vi "画箭头.vi"(0 "Image 2":T1(plugin-control)=refnum, 5 "距离":dbl, 7 "Rectangle":T3={"Left"=1066, "Top"=296, "Right"=344, "Bottom"=354, "Rotation"=45.0} {"Rotation" format="%.2f"; "Left" scale=0.0..1024.0; "Right" scale=0.0..1024.0}, 9 "abgek":dbl, 11 "error in (no error)":errorcluster caption="错误输入（无错误）", 12 "long":sgl=15.0, 13 "Color 2":u32(colorbox)=16711680) -> (4 "Image":T1(plugin-control), 15 "error out":errorcluster)   [LabVIEW 2017]
uses:
  <vilib>/Analysis/coordinate.llb/2D Cartesian Coordinate Shift (Array).vi
  <vilib>/Analysis/coordinate.llb/2D Cartesian Coordinate Rotation (Array).vi
  <vilib>/Analysis/NI_AALPro.lvlib
panel:
  out "下":dbl
  out "上":dbl
  in  "Width":u32=23
  out "添加的数组":T2[](array[typedef]) {"Y" format="%.2f"; "X" format="%.2f"}
  in  "Color":u32(colorbox)=16711680
  out "MiddleEndPoint":T2={"X"=892.0, "Y"=1299.75} {"Y" format="%.2f"; "X" format="%.2f"}
  out "MiddleStartPoint":T2={"X"=892.0, "Y"=1159.25} {"Y" format="%.2f"; "X" format="%.2f"}
  out "EndPoint":T2={"X"=892.0, "Y"=1370.0} {"Y" format="%.2f"; "X" format="%.2f"}
  out "StartPoint":T2={"X"=892.0, "Y"=1089.0} {"Y" format="%.2f"; "X" format="%.2f"}
  in  "sss":i32=30
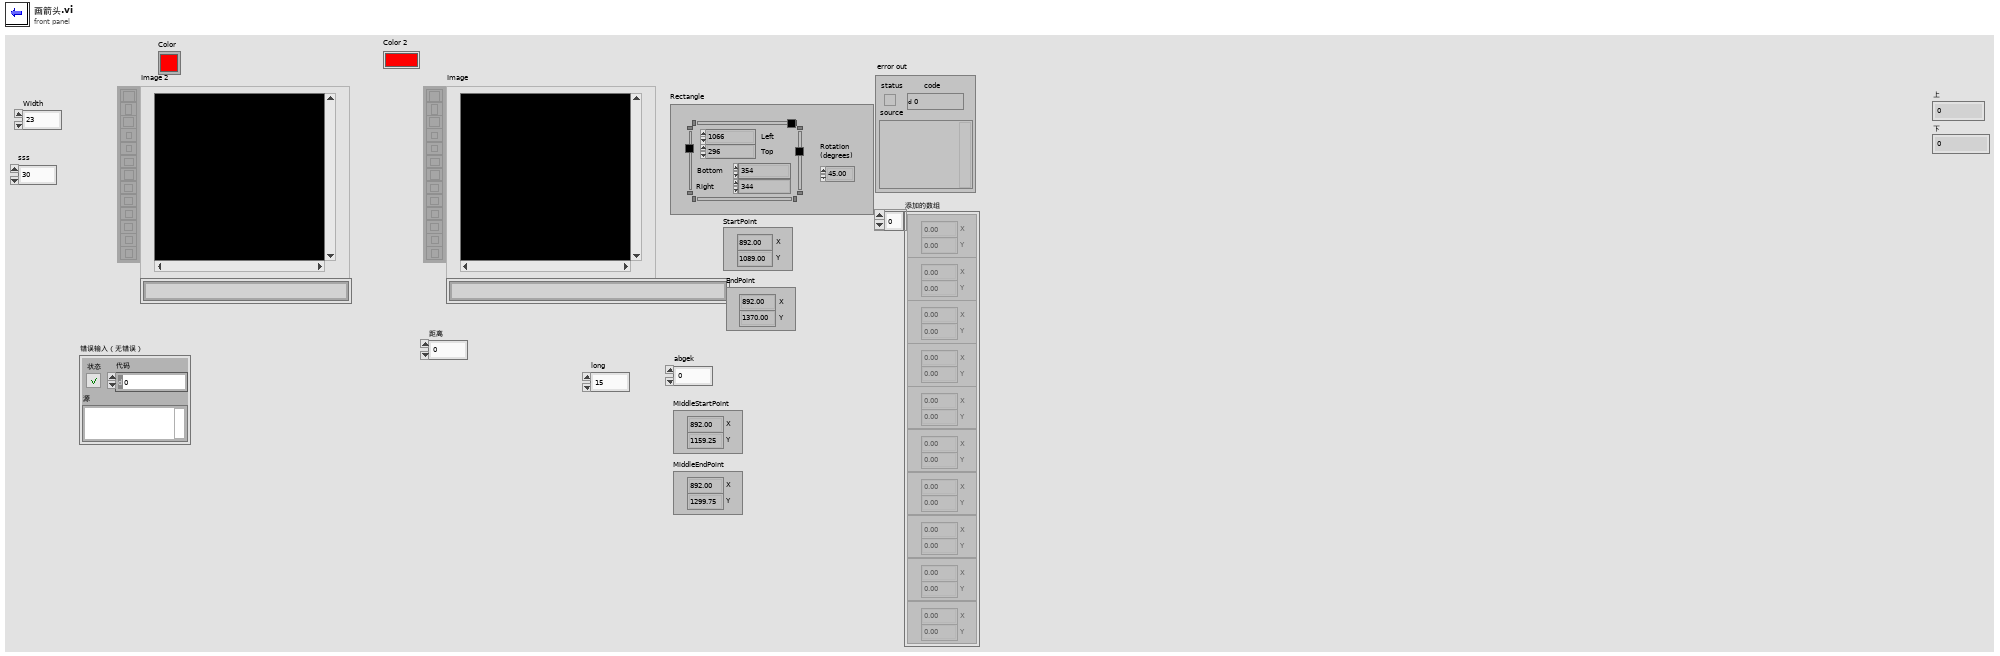
[diagram p1: front panel]
types:
  T1 = typedef "IMAQ Image.ctl" = refnum<image>
  T2 = typedef "IMAQ Point" = cluster{"X":sgl, "Y":sgl}
  T3 = typedef "IMAQ Rectangle" = cluster{"Left":i32, "Top":i32, "Right":i32, "Bottom":i32, "Rotation":dbl}
  T4 = cluster{"Desired Font (Application)":enum16{"User-specified Font", "Application Font", "System Font", "Dialog Font"}, "[User-specified Font]":cluster{"Font Name":string, "Size":i16, "Strikeout?":bool, "Italic?":bool, "Underline?":bool, "Outline?":bool, "Shadow?":bool, "Bold?":bool, "Rotation Angle":dbl}, "Horizontal Alignment":i16, "Vertical Alignment":i16}
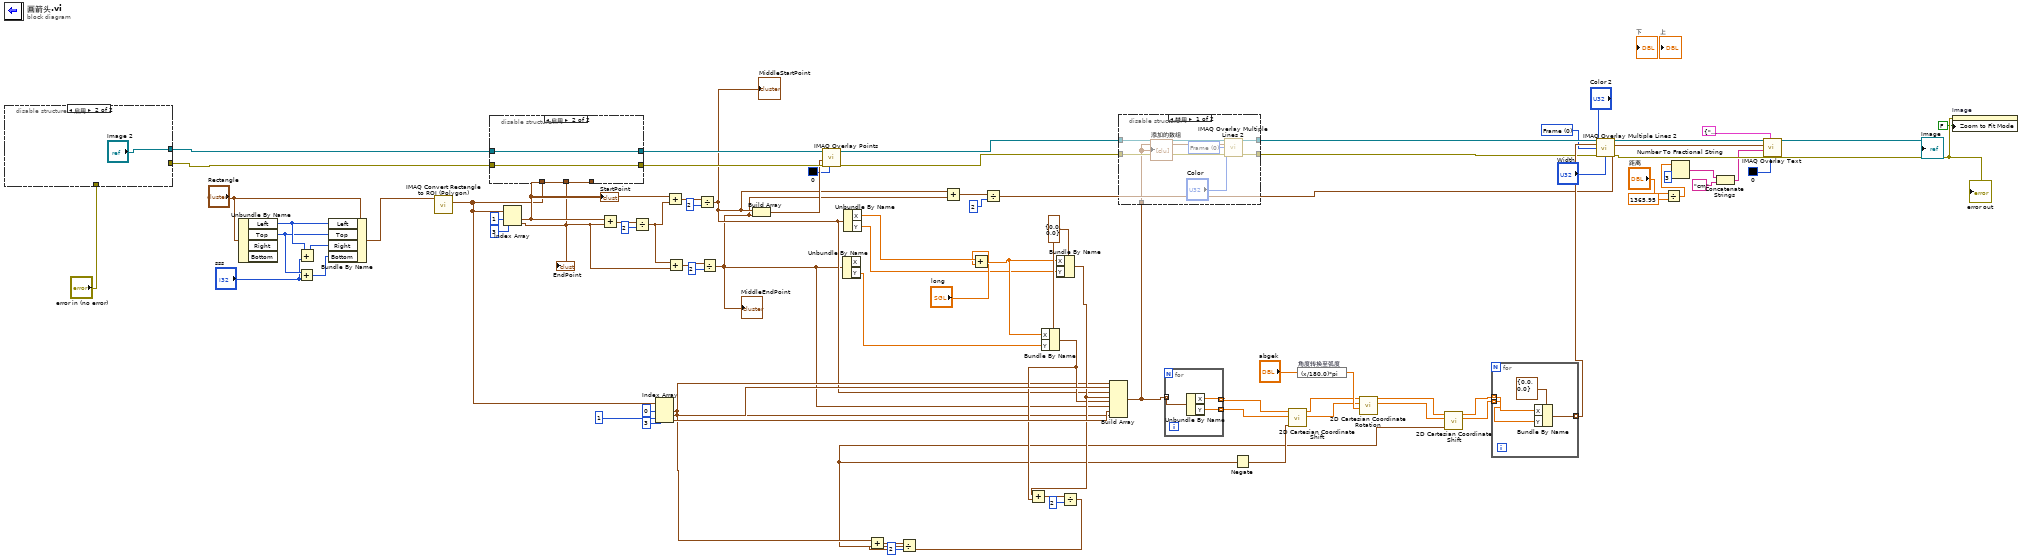
[diagram p0: block diagram]
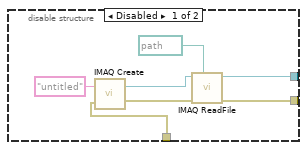
[diagram p2: hidden frame]
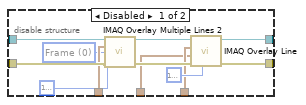
[diagram p4: hidden frame]
diagram:
  w32 = u32 0 items=["Frame", "Fill"] ("Drawing Mode (Frame)")
  w54 = T2 {"X"=0.0, "Y"=0.0} ("元素")
  n1 = disable-structure shown="启用" {
    disable-tunnel: [w87 "Image 2"] -> w17
    disable-tunnel: [w86 _] -> w16
    disable-tunnel: "error in (no error)" -> [w85 _]
    frame Disabled {
      n2 = call "IMAQ Create"("Image Name"="untitled", "error in (no error)"=w85) -> ("New Image"=w89:T1, "error out"=w90:errorcluster)  [unwired: 3 in]
      n3 = call "IMAQ ReadFile"("File Path"=path "C:/Users/Lenovo/Desktop/PowerLine Inspect System/微信图片_20181113103336.bmp", "error in (no error)"=w90, "Image"=w89) -> ("error out"=w86:errorcluster, "Image Out"=w87:T1)  [unwired: 4 in, 3 out]
    }
    frame Enabled {
    }
  }
  n4 = Unbundle By Name("Rectangle") -> ("Left"=w82:i32, "Top"=w80:i32)  [unwired: 2 out]
  n5 = Add(x=w80, y="sss") -> (x+y=w78:i32)
  n6 = Add(x=w82, y="sss") -> (x+y=w81:i32)
  n7 = Bundle By Name(cluster="Rectangle", "Left"=w82, "Top"=w80, "Right"=w81, "Bottom"=w78) -> (w83:T3)
  n8 = call "IMAQ Convert Rectangle to ROI (Polygon)"("Rectangle"=w83) -> ("Rectangle Points"=w57:T2[])  [unwired: 7 in, 2 out]
  n9 = Index Array(array=w57, index #1=1 ("索引"), index #2=3 ("索引")) -> (element #1=w70:T2, element #2=w66:T2)
  "StartPoint" <- w70
  "EndPoint" <- w66
  n10 = disable-structure shown="启用" {
    disable-tunnel: w17 -> [w103 w106]
    disable-tunnel: w16 -> [w102 w105]
    disable-tunnel: [w101 w106] -> w77
    disable-tunnel: w70 -> [w98 _]
    disable-tunnel: w66 -> [w97 _]
    disable-tunnel: [w96 w105] -> w64
    disable-tunnel: w57 -> [w95 _]
    frame Disabled {
      w94 = u32 0 items=["Frame", "Fill"] ("Drawing Mode (Frame)")
      n11 = call "IMAQ Overlay Multiple Lines 2"("Image"=w103, "Line End Points"=w95, "Drawing Mode (Frame)"=w94, "Color"=u32 16777238, "error in (no error)"=w102) -> ("Image Out"=w104:T1, "error out"=w100:errorcluster)  [unwired: 9 in]
      n12 = call "IMAQ Overlay Line"("Color"=u32 16777238, "error in (no error)"=w100, "End Point"=w97, "Start Point"=w98, "Image"=w104) -> ("error out"=w96:errorcluster, "Image Out"=w101:T1)  [unwired: 5 in]
    }
    frame Enabled {
    }
  }
  n13 = Add(x=w70, y=w66) -> (x+y=w74:T2)
  n14 = Divide(x=w74, y=2) -> (x/y=w67:T2)
  n15 = Index Array(array=w57, index #1=0 ("索引"), index #2=1 ("索引"), index #3=3 ("索引")) -> (element #1=w24:T2, element #2=w56:T2, element #3=w48:T2)
  n16 = Add(x=w70, y=w67) -> (x+y=w71:T2)
  n17 = Add(x=w67, y=w66) -> (x+y=w69:T2)
  n18 = Divide(x=w71, y=2) -> (x/y=w11:T2)
  "MiddleStartPoint" <- w11
  n19 = Divide(x=w69, y=2) -> (x/y=w10:T2)
  "MiddleEndPoint" <- w10
  n20 = Build Array(w11, w10) -> (w63:T2[])
  n21 = call "IMAQ Overlay Points"("Color"=u32 0, "error in (no error)"=w64, "Array of Points"=w63, "Image"=w77) -> ("error out"=w60:errorcluster, "Image Out"=w65:T1)  [unwired: 6 in]
  n22 = Unbundle By Name(w10) -> ("Y"=w50:sgl)  [unwired: 1 out]
  n23 = Unbundle By Name(w11) -> ("X"=w55:sgl, "Y"=w51:sgl)
  n24 = Add(x=w11, y=w10) -> (x+y=w9:T2)
  n25 = Add(x=w55, y="long") -> (x+y=w53:sgl)
  n26 = Divide(x=w9, y=2) -> (x/y=w7:T2)
  n27 = Bundle By Name(cluster=w54, "X"=w53, "Y"=w50) -> (w26:T2)
  n28 = Bundle By Name(cluster=w54, "X"=w53, "Y"=w51) -> (w27:T2)
  n29 = Add(x=w27, y=w26) -> (x+y=w28:T2)
  n30 = Divide(x=w28, y=2) -> (x/y=w25:T2)
  n31 = Add(x=w24, y=w25) -> (x+y=w31:T2)
  n32 = Divide(x=w31, y=2) -> (x/y=w23:T2)
  n33 = Build Array(w24, w56, w11, w27, w26, w10, w48, w24) -> (w47:T2[])
  n34 = disable-structure shown="禁用" {
    disable-tunnel: w65 -> [w113 w115]
    disable-tunnel: [w112 w115] -> w61
    disable-tunnel: w60 -> [w111 w114]
    disable-tunnel: w47 -> [w110 _]
    disable-tunnel: [w109 w114] -> w42
    frame Disabled {
      w107 = u32 0 items=["Frame", "Fill"] ("Drawing Mode (Frame)")
      n35 = call "IMAQ Overlay Multiple Lines 2"("Image"=w113, "Line End Points"=w110, "Drawing Mode (Frame)"=w107, "Color"="Color", "error in (no error)"=w111) -> ("Image Out"=w112:T1, "error out"=w109:errorcluster)  [unwired: 9 in]
      "添加的数组" <- w110
    }
    frame Enabled {
    }
  }
  n36 = for {
    tunnel: w47 -> [w118] mode=indexing
    tunnel: [w117] -> w41 mode=indexing
    tunnel: [w116] -> w40 mode=indexing
    n37 = Unbundle By Name(w118) -> ("X"=w117:sgl, "Y"=w116:sgl)
  }
  n38 = Negate(x=w23) -> (-x=w39:T2)
  n39 = call-poly <vilib>:"2D Cartesian Coordinate Shift.vi"("shift"=w39, "Y"=w40, "X"=w41) -> ("Y Out"=w37:dbl[], "X Out"=w38:dbl[])  [unwired: 6 in, 1 out]
  n40 = expression code="(x/180.0)*pi" "角度转换至弧度"("abgek") -> (w45:dbl)
  n41 = call-poly <vilib>:"2D Cartesian Coordinate Rotation.vi"("theta"=w45, "Y"=w37, "X"=w38) -> ("Y Out"=w34:dbl[], "X Out"=w36:dbl[])  [unwired: 6 in, 1 out]
  n42 = call-poly <vilib>:"2D Cartesian Coordinate Shift.vi"("shift"=w23, "Y"=w34, "X"=w36) -> ("Y Out"=w33:dbl[], "X Out"=w35:dbl[])  [unwired: 6 in, 1 out]
  n43 = for {
    tunnel: w35 -> [w121] mode=indexing
    tunnel: w33 -> [w120] mode=indexing
    tunnel: [w119] -> w43 mode=indexing
    n44 = Bundle By Name(cluster=T2 {"X"=0.0, "Y"=0.0} ("元素"), "X"=w121, "Y"=w120) -> (w119:T2)
  }
  n45 = call "IMAQ Overlay Multiple Lines 2"("Image"=w61, "Line End Points"=w43, "Drawing Mode (Frame)"=w32, "Color"="Color 2", "error in (no error)"=w42, "Width"="Width") -> ("Image Out"=w44:T1, "error out"=w21:errorcluster)  [unwired: 8 in]
  "error out" <- w21
  n46 = Divide(x="距离", y=1365.95) -> (x/y=w4:dbl)
  n47 = Number To Fractional String(number=w4, precision (6)=i16 3 ("精度(6)")) -> (F-format string=w3:string)  [unwired: 2 in]
  n48 = Concatenate Strings(w3, "cm" ("元素")) -> (w1:string)
  n49 = call "IMAQ Overlay Text"("Text Color (black)"=u32 0, "Font, Size & Style"=T4 {"Desired Font (Application)"=enum."User-specified Font", "[User-specified Font]"={"Font Name"="", "Size"=15, "Strikeout?"=FALSE, "Italic?"=FALSE, "Underline?"=FALSE, "Outline?"=FALSE, "Shadow?"=FALSE, "Bold?"=TRUE, "Rotation Angle"=0.0}, "Horizontal Alignment"=1, "Vertical Alignment"=0}, "String"=w1, "Origin"=w7, "Image"=w44) -> ("Image Out"=→"Image":T1)  [unwired: 5 in, 1 out]
  n50 = property on="Image" class="ImageControl"(error in=w21, "Zoom to Fit Mode"=FALSE) -> ()  [unwired: 1 in, 2 out]
